vi "s.vi"() -> ()   [LabVIEW 2013] (continued)
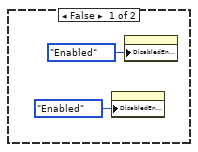
[diagram p2: hidden frame]
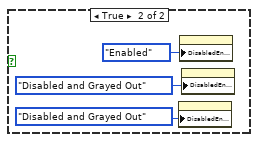
[diagram p3: hidden frame]
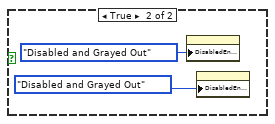
[diagram p4: hidden frame]
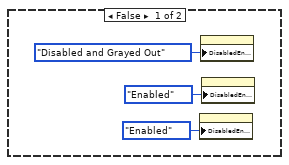
[diagram p5: hidden frame]
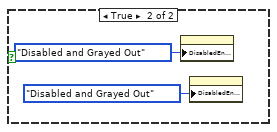
[diagram p6: hidden frame]
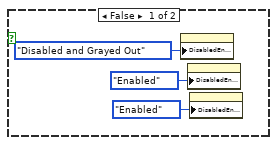
[diagram p7: hidden frame]
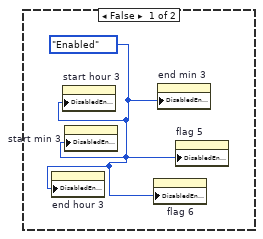
[diagram p8: hidden frame]
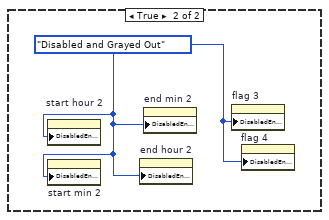
[diagram p9: hidden frame]
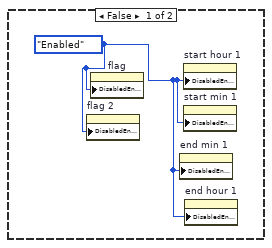
[diagram p10: hidden frame]
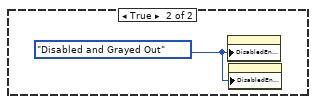
[diagram p11: hidden frame]
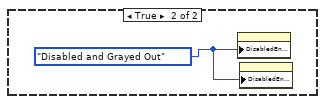
[diagram p12: hidden frame]
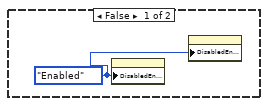
[diagram p13: hidden frame]
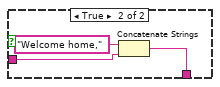
[diagram p16: hidden frame]
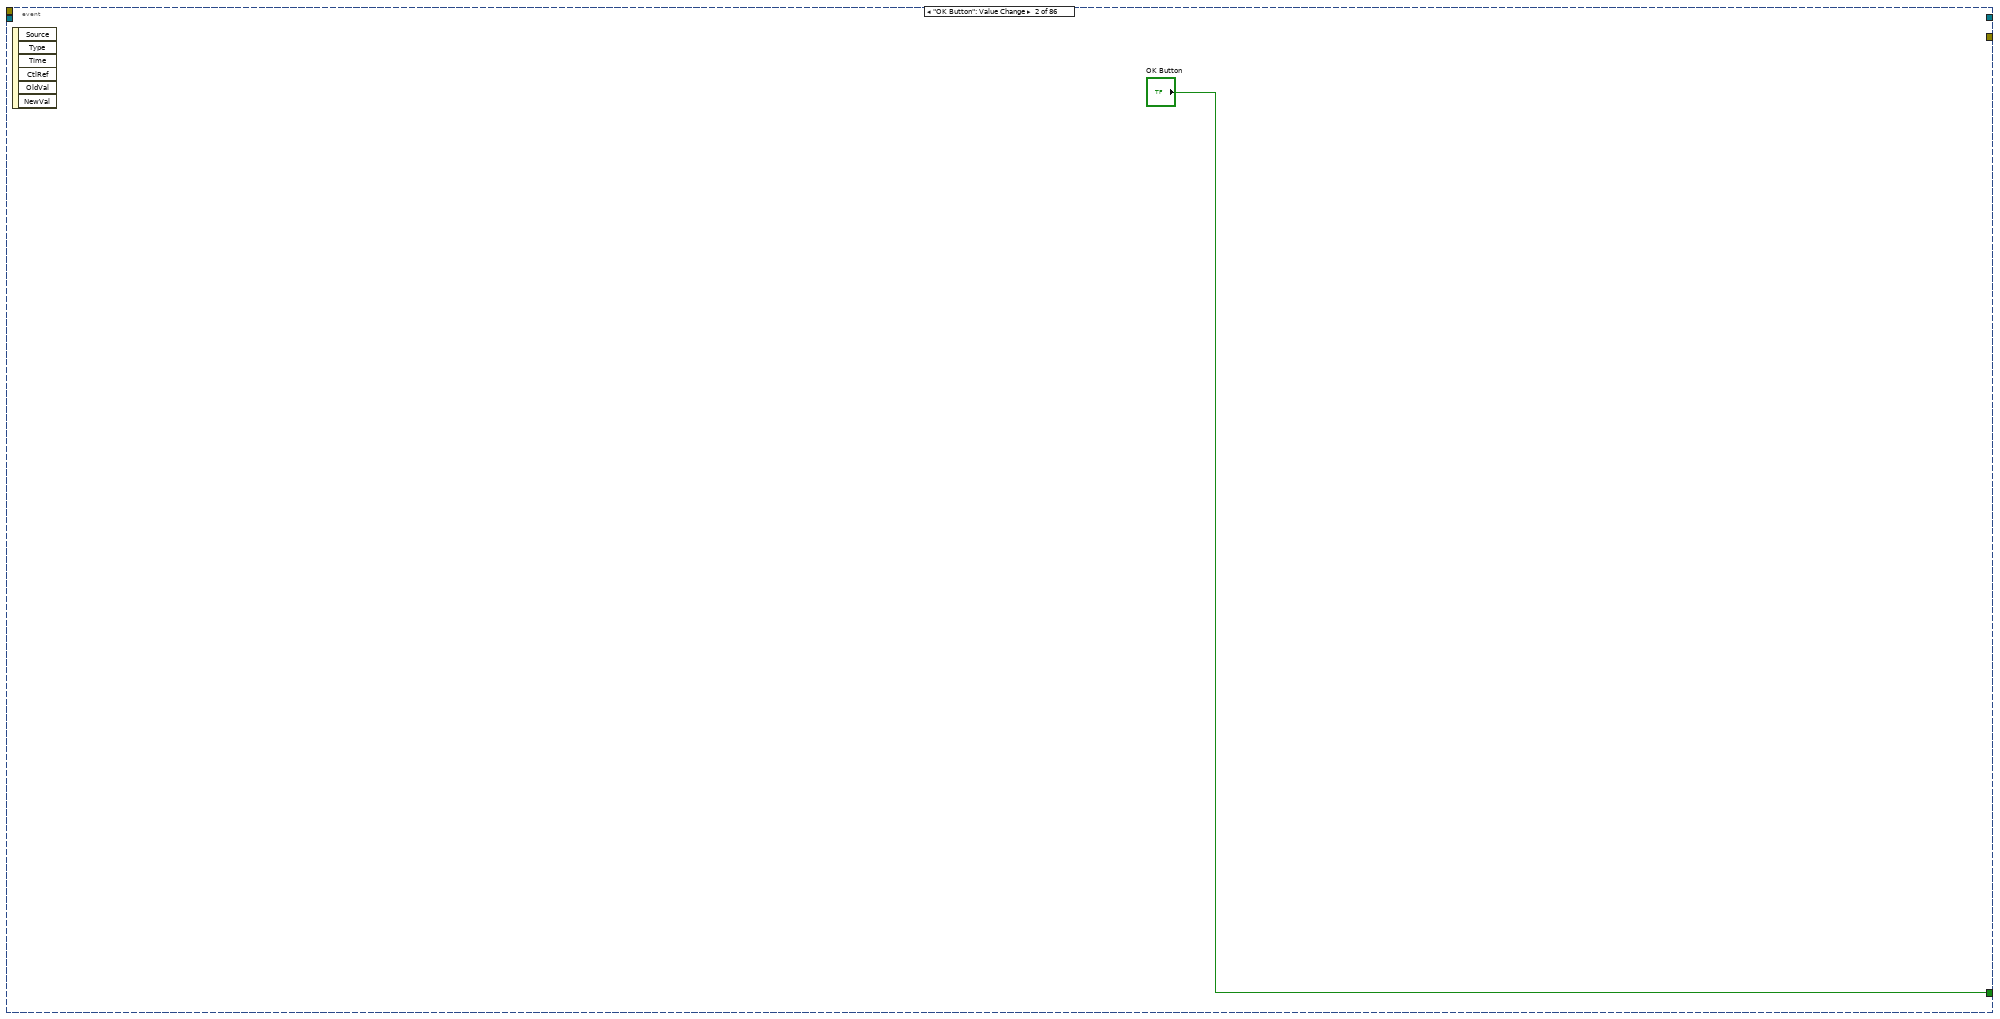
[diagram p17: hidden frame]
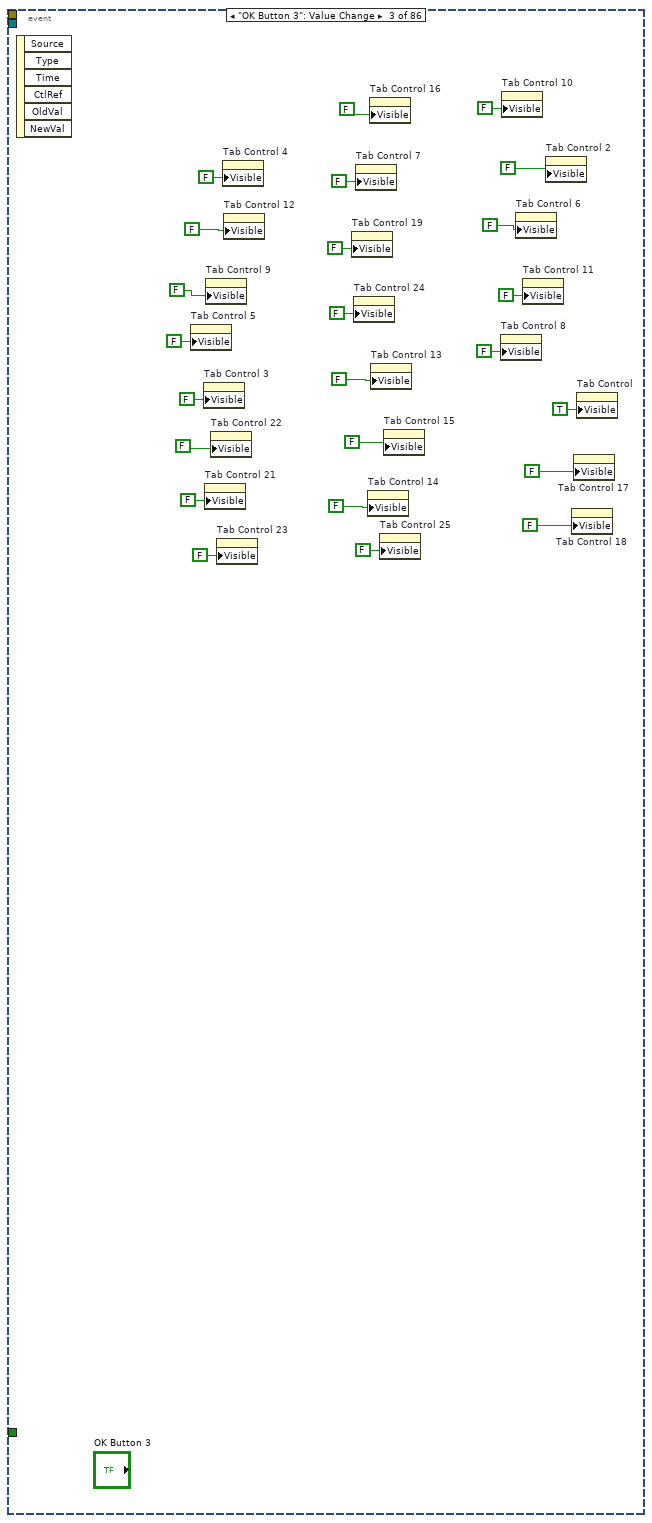
[diagram p18: hidden frame]
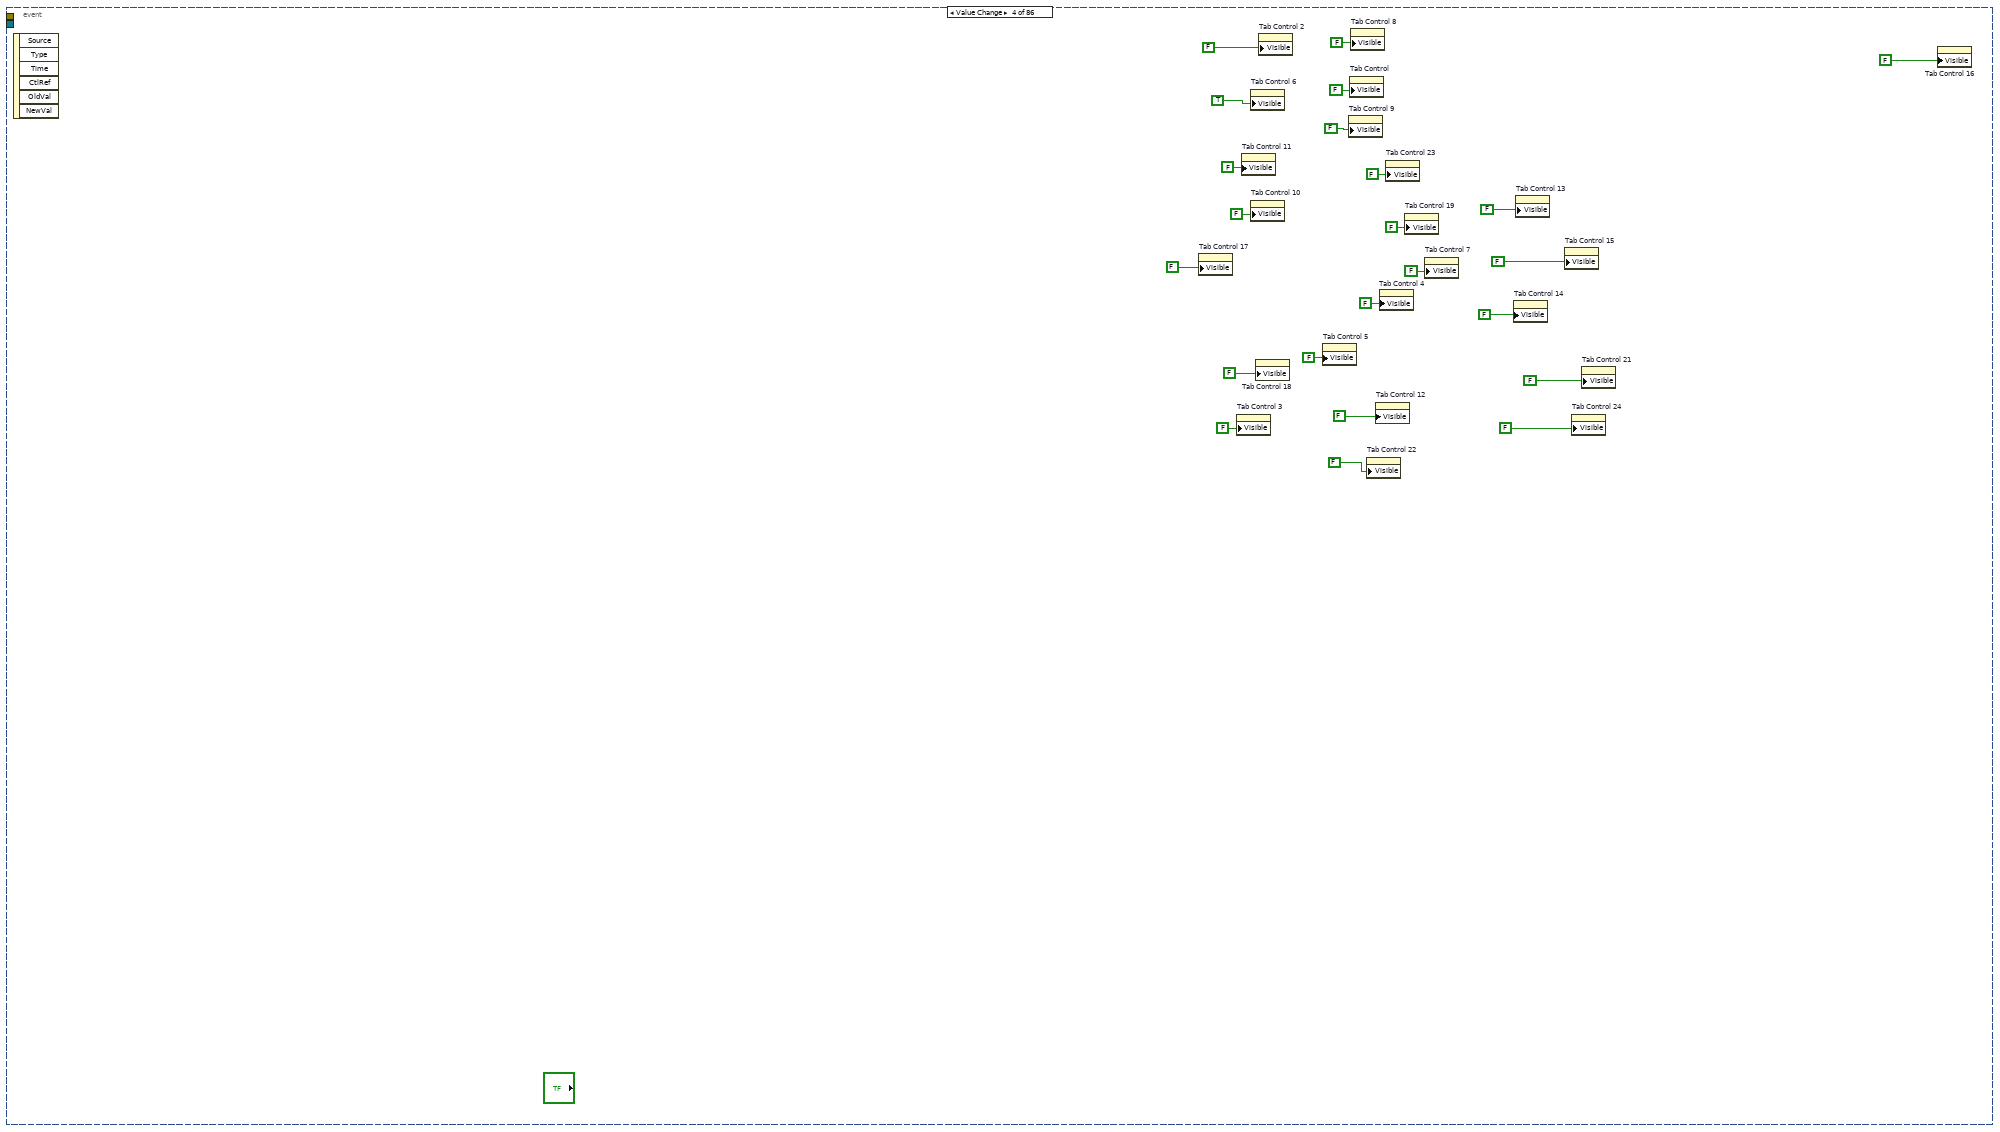
[diagram p19: hidden frame]
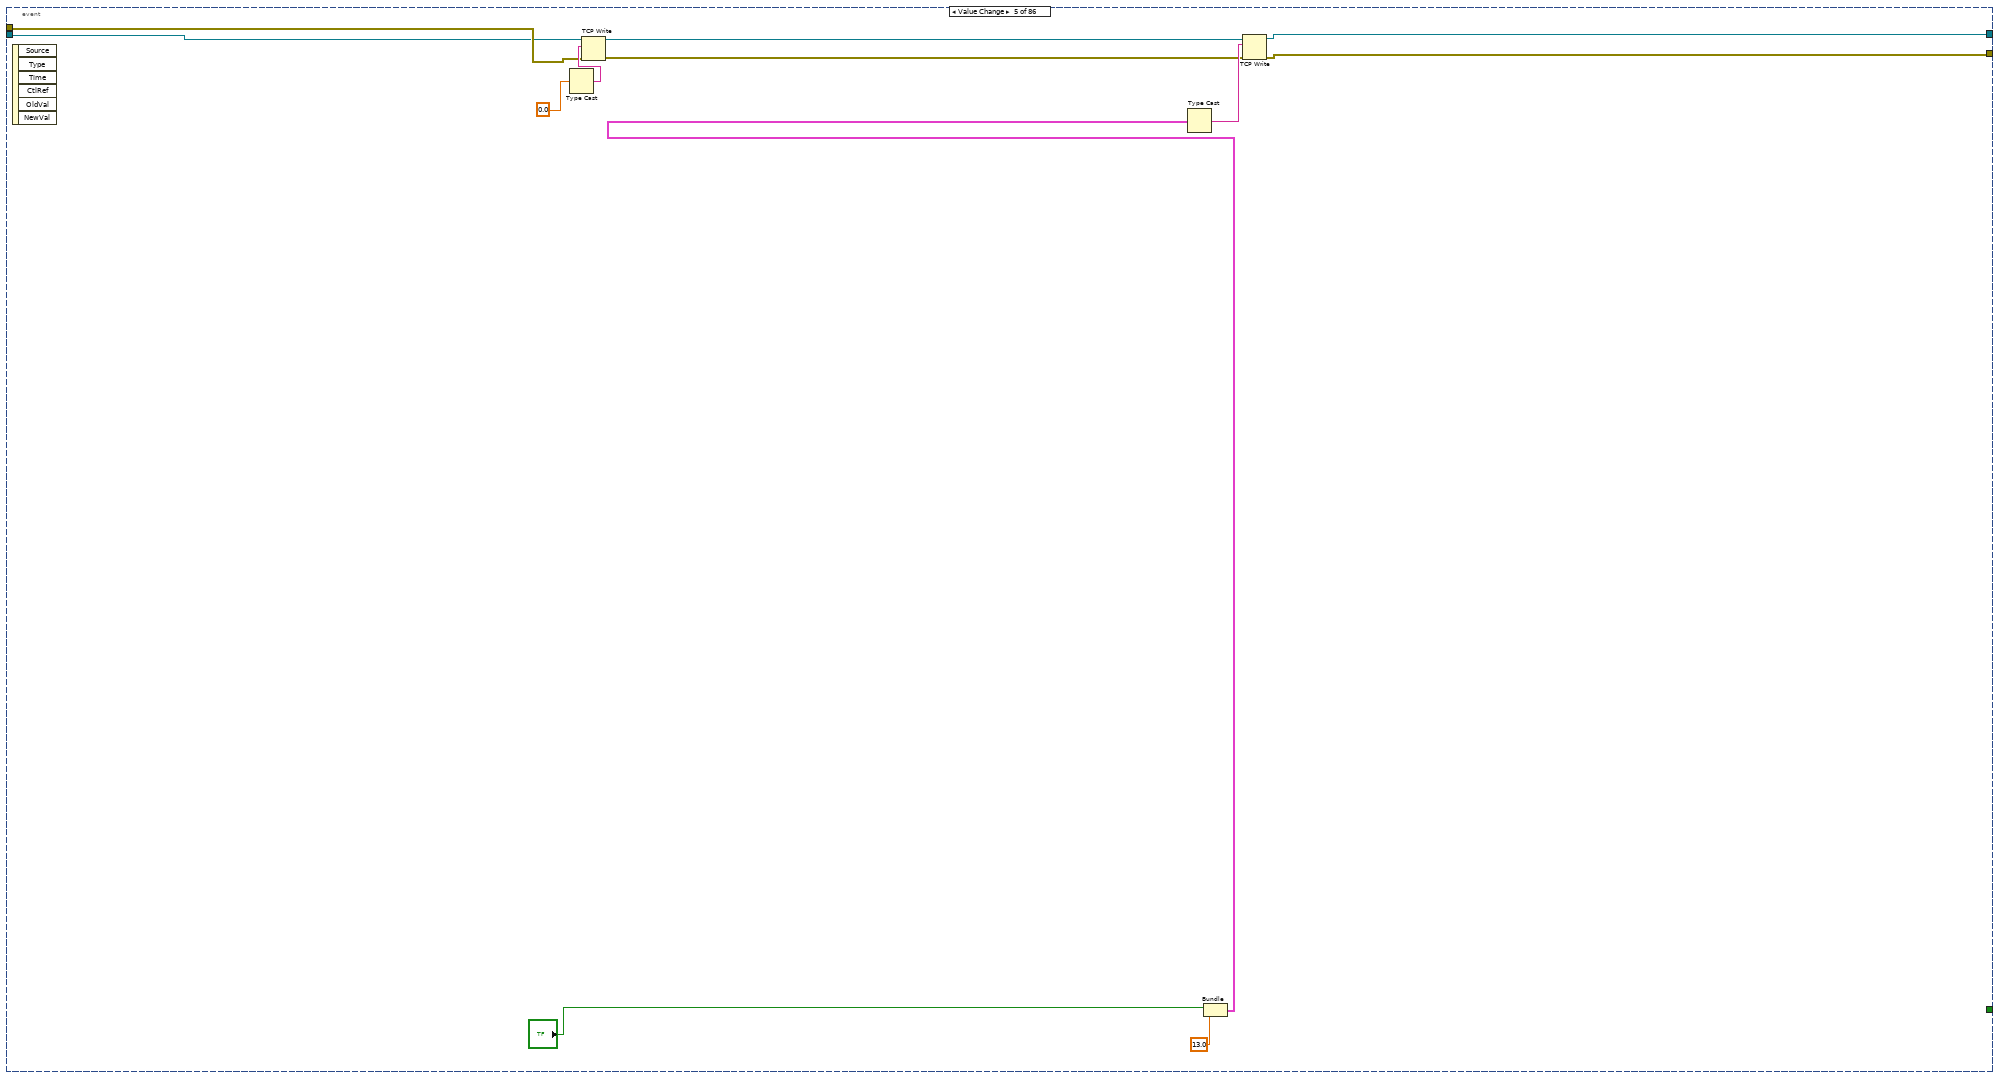
[diagram p20: hidden frame]
        n991 = property on="Tab Control 15" class="TabCtl (strict)"("Visible"=FALSE) -> ()  [unwired: 2 in, 2 out]
        n992 = property on="Tab Control 16" class="TabCtl (strict)"("Visible"=FALSE) -> ()  [unwired: 2 in, 2 out]
        n993 = property on="Tab Control 17" class="TabCtl (strict)"("Visible"=FALSE) -> ()  [unwired: 2 in, 2 out]
        n994 = property on="Tab Control 21" class="TabCtl (strict)"("Visible"=FALSE) -> ()  [unwired: 2 in, 2 out]
        n995 = property on="Tab Control 18" class="TabCtl (strict)"("Visible"=FALSE) -> ()  [unwired: 2 in, 2 out]
        n996 = property on="Tab Control 24" class="TabCtl (strict)"("Visible"=FALSE) -> ()  [unwired: 2 in, 2 out]
        n997 = property on="Tab Control 19" class="TabCtl (strict)"("Visible"=TRUE) -> ()  [unwired: 2 in, 2 out]
        n998 = property on="Tab Control 22" class="TabCtl (strict)"("Visible"=FALSE) -> ()  [unwired: 2 in, 2 out]
      }
      event "OK Button 6": Value Change {
        n999 = event-data() -> ()  [unwired: 1 in, 6 out]
        n1000 = Type Cast(x=0.0) -> (*(type *) &x=w3067:string)  [unwired: 1 in]
        n1001 = TCP Write(connection ID=w3065, data in=w3067, error in (no error)=w3066) -> (connection ID out=w3064:refnum<k5>, error out=w3063:errorcluster)  [unwired: 1 in, 1 out]
        n1002 = Bundle("OK Button 6"="OK Button 6", 5.0) -> (w3072:cluster{"OK Button 6":bool, dbl})  [unwired: 1 in]
        n1003 = Type Cast(x=w3072) -> (*(type *) &x=w3073:string)  [unwired: 1 in]
        n1004 = TCP Write(connection ID=w3064, data in=w3073, error in (no error)=w3063) -> (connection ID out=w3069:refnum<k5>, error out=w3070:errorcluster)  [unwired: 1 in, 1 out]
      }
      event Value Change {
        # "Air conditional - Master room"
        n1005 = event-data() -> ()  [unwired: 1 in, 6 out]
        n1006 = property on="Tab Control" class="TabCtl (strict)"("Visible"=FALSE) -> ()  [unwired: 2 in, 2 out]
        n1007 = property on="Tab Control 2" class="TabCtl (strict)"("Visible"=FALSE) -> ()  [unwired: 2 in, 2 out]
        n1008 = property on="Tab Control 3" class="TabCtl (strict)"("Visible"=FALSE) -> ()  [unwired: 2 in, 2 out]
        n1009 = property on="Tab Control 4" class="TabCtl (strict)"("Visible"=FALSE) -> ()  [unwired: 2 in, 2 out]
        n1010 = property on="Tab Control 5" class="TabCtl (strict)"("Visible"=FALSE) -> ()  [unwired: 2 in, 2 out]
        n1011 = property on="Tab Control 13" class="TabCtl (strict)"("Visible"=FALSE) -> ()  [unwired: 2 in, 2 out]
        n1012 = property on="Tab Control 14" class="TabCtl (strict)"("Visible"=FALSE) -> ()  [unwired: 2 in, 2 out]
        n1013 = property on="Tab Control 11" class="TabCtl (strict)"("Visible"=FALSE) -> ()  [unwired: 2 in, 2 out]
        n1014 = property on="Tab Control 6" class="TabCtl (strict)"("Visible"=FALSE) -> ()  [unwired: 2 in, 2 out]
        n1015 = property on="Tab Control 10" class="TabCtl (strict)"("Visible"=FALSE) -> ()  [unwired: 2 in, 2 out]
        n1016 = property on="Tab Control 7" class="TabCtl (strict)"("Visible"=FALSE) -> ()  [unwired: 2 in, 2 out]
        n1017 = property on="Tab Control 12" class="TabCtl (strict)"("Visible"=FALSE) -> ()  [unwired: 2 in, 2 out]
        n1018 = property on="Tab Control 8" class="TabCtl (strict)"("Visible"=FALSE) -> ()  [unwired: 2 in, 2 out]
        n1019 = property on="Tab Control 9" class="TabCtl (strict)"("Visible"=FALSE) -> ()  [unwired: 2 in, 2 out]
        n1020 = property on="Tab Control 15" class="TabCtl (strict)"("Visible"=FALSE) -> ()  [unwired: 2 in, 2 out]
        n1021 = property on="Tab Control 16" class="TabCtl (strict)"("Visible"=FALSE) -> ()  [unwired: 2 in, 2 out]
        n1022 = property on="Tab Control 17" class="TabCtl (strict)"("Visible"=FALSE) -> ()  [unwired: 2 in, 2 out]
        n1023 = property on="Tab Control 24" class="TabCtl (strict)"("Visible"=FALSE) -> ()  [unwired: 2 in, 2 out]
        n1024 = property on="Tab Control 18" class="TabCtl (strict)"("Visible"=FALSE) -> ()  [unwired: 2 in, 2 out]
        n1025 = property on="Tab Control 21" class="TabCtl (strict)"("Visible"=FALSE) -> ()  [unwired: 2 in, 2 out]
        n1026 = property on="Tab Control 19" class="TabCtl (strict)"("Visible"=FALSE) -> ()  [unwired: 2 in, 2 out]
        n1027 = property on="Tab Control 22" class="TabCtl (strict)"("Visible"=TRUE) -> ()  [unwired: 2 in, 2 out]
      }
      event Value Change {
        # "Air conditional - Bedroom 1"
        n1028 = event-data() -> ()  [unwired: 1 in, 6 out]
        n1029 = property on="Tab Control" class="TabCtl (strict)"("Visible"=FALSE) -> ()  [unwired: 2 in, 2 out]
        n1030 = property on="Tab Control 2" class="TabCtl (strict)"("Visible"=FALSE) -> ()  [unwired: 2 in, 2 out]
        n1031 = property on="Tab Control 3" class="TabCtl (strict)"("Visible"=FALSE) -> ()  [unwired: 2 in, 2 out]
        n1032 = property on="Tab Control 4" class="TabCtl (strict)"("Visible"=FALSE) -> ()  [unwired: 2 in, 2 out]
        n1033 = property on="Tab Control 5" class="TabCtl (strict)"("Visible"=FALSE) -> ()  [unwired: 2 in, 2 out]
        n1034 = property on="Tab Control 11" class="TabCtl (strict)"("Visible"=FALSE) -> ()  [unwired: 2 in, 2 out]
        n1035 = property on="Tab Control 6" class="TabCtl (strict)"("Visible"=FALSE) -> ()  [unwired: 2 in, 2 out]
        n1036 = property on="Tab Control 10" class="TabCtl (strict)"("Visible"=FALSE) -> ()  [unwired: 2 in, 2 out]
        n1037 = property on="Tab Control 13" class="TabCtl (strict)"("Visible"=FALSE) -> ()  [unwired: 2 in, 2 out]
        n1038 = property on="Tab Control 7" class="TabCtl (strict)"("Visible"=FALSE) -> ()  [unwired: 2 in, 2 out]
        n1039 = property on="Tab Control 12" class="TabCtl (strict)"("Visible"=FALSE) -> ()  [unwired: 2 in, 2 out]
        n1040 = property on="Tab Control 8" class="TabCtl (strict)"("Visible"=FALSE) -> ()  [unwired: 2 in, 2 out]
        n1041 = property on="Tab Control 9" class="TabCtl (strict)"("Visible"=FALSE) -> ()  [unwired: 2 in, 2 out]
        n1042 = property on="Tab Control 21" class="TabCtl (strict)"("Visible"=FALSE) -> ()  [unwired: 2 in, 2 out]
        n1043 = property on="Tab Control 22" class="TabCtl (strict)"("Visible"=FALSE) -> ()  [unwired: 2 in, 2 out]
        n1044 = property on="Tab Control 23" class="TabCtl (strict)"("Visible"=TRUE) -> ()  [unwired: 2 in, 2 out]
        n1045 = property on="Tab Control 24" class="TabCtl (strict)"("Visible"=FALSE) -> ()  [unwired: 2 in, 2 out]
        n1046 = property on="Tab Control 14" class="TabCtl (strict)"("Visible"=FALSE) -> ()  [unwired: 2 in, 2 out]
        n1047 = property on="Tab Control 15" class="TabCtl (strict)"("Visible"=FALSE) -> ()  [unwired: 2 in, 2 out]
        n1048 = property on="Tab Control 20" class="TabCtl (strict)"("Visible"=FALSE) -> ()  [unwired: 2 in, 2 out]
        n1049 = property on="Tab Control 16" class="TabCtl (strict)"("Visible"=FALSE) -> ()  [unwired: 2 in, 2 out]
        n1050 = property on="Tab Control 17" class="TabCtl (strict)"("Visible"=FALSE) -> ()  [unwired: 2 in, 2 out]
        n1051 = property on="Tab Control 18" class="TabCtl (strict)"("Visible"=FALSE) -> ()  [unwired: 2 in, 2 out]
        n1052 = property on="Tab Control 19" class="TabCtl (strict)"("Visible"=FALSE) -> ()  [unwired: 2 in, 2 out]
      }
      event "OK Button 7": Value Change {
        n1053 = event-data() -> ()  [unwired: 1 in, 6 out]
        n1054 = Type Cast(x=0.0) -> (*(type *) &x=w3125:string)  [unwired: 1 in]
        n1055 = TCP Write(connection ID=w3123, data in=w3125, error in (no error)=w3120) -> (connection ID out=w3122:refnum<k5>, error out=w3121:errorcluster)  [unwired: 1 in, 1 out]
        n1056 = Bundle("OK Button 7"="OK Button 7", 6.0) -> (w3130:cluster{"OK Button 7":bool, dbl})  [unwired: 1 in]
        n1057 = Type Cast(x=w3130) -> (*(type *) &x=w3131:string)  [unwired: 1 in]
        n1058 = TCP Write(connection ID=w3122, data in=w3131, error in (no error)=w3121) -> (connection ID out=w3127:refnum<k5>, error out=w3128:errorcluster)  [unwired: 1 in, 1 out]
      }
      event "OK Button 8": Value Change {
        n1059 = event-data() -> ()  [unwired: 1 in, 6 out]
        n1060 = Type Cast(x=0.0) -> (*(type *) &x=w3137:string)  [unwired: 1 in]
        n1061 = TCP Write(connection ID=w3133, data in=w3137, error in (no error)=w3132) -> (connection ID out=w3134:refnum<k5>, error out=w3135:errorcluster)  [unwired: 1 in, 1 out]
        n1062 = Bundle("OK Button 8"="OK Button 8", 7.0) -> (w3142:cluster{"OK Button 8":bool, dbl})  [unwired: 1 in]
        n1063 = Type Cast(x=w3142) -> (*(type *) &x=w3143:string)  [unwired: 1 in]
        n1064 = TCP Write(connection ID=w3134, data in=w3143, error in (no error)=w3135) -> (connection ID out=w3139:refnum<k5>, error out=w3140:errorcluster)  [unwired: 1 in, 1 out]
      }
      event "OK Button 9": Value Change {
        n1065 = event-data() -> ()  [unwired: 1 in, 6 out]
        n1066 = Type Cast(x=0.0) -> ()  [unwired: 1 in, 1 out]
        n1067 = TCP Write(connection ID=w3145, error in (no error)=w3144) -> (connection ID out=w3146:refnum<k5>, error out=w3147:errorcluster)  [unwired: 2 in, 1 out]
        n1068 = Bundle("OK Button 9"="OK Button 9", 10.0) -> (w3153:cluster{"OK Button 9":bool, dbl})  [unwired: 1 in]
        n1069 = Type Cast(x=w3153) -> (*(type *) &x=w3154:string)  [unwired: 1 in]
        n1070 = TCP Write(connection ID=w3146, data in=w3154, error in (no error)=w3147) -> (connection ID out=w3150:refnum<k5>, error out=w3151:errorcluster)  [unwired: 1 in, 1 out]
      }
      event "OK Button 10": Value Change {
        n1071 = event-data() -> ()  [unwired: 1 in, 6 out]
        n1072 = Type Cast(x=0.0) -> ()  [unwired: 1 in, 1 out]
        n1073 = TCP Write(connection ID=w3158, error in (no error)=w3157) -> (connection ID out=w3156:refnum<k5>, error out=w3155:errorcluster)  [unwired: 2 in, 1 out]
        n1074 = Bundle("OK Button 10"="OK Button 10", 11.0) -> (w3164:cluster{"OK Button 10":bool, dbl})  [unwired: 1 in]
        n1075 = Type Cast(x=w3164) -> (*(type *) &x=w3165:string)  [unwired: 1 in]
        n1076 = TCP Write(connection ID=w3156, data in=w3165, error in (no error)=w3155) -> (connection ID out=w3161:refnum<k5>, error out=w3162:errorcluster)  [unwired: 1 in, 1 out]
      }
    }
    n1077 = case shown="True" w28 {
      frame False {
        w75 = T1."Enabled" ("Disabled")
        n1078 = property class="Slide (strict)"("DisabledEnum"=w75) -> ()  [unwired: 2 in, 2 out]
        n1079 = property class="Str"("DisabledEnum"=w75) -> ()  [unwired: 2 in, 2 out]
      }
      frame True {
        w76 = T1."Disabled and Grayed Out" ("Disabled")
        n1080 = property class="Slide (strict)"("DisabledEnum"=w76) -> ()  [unwired: 2 in, 2 out]
        n1081 = property class="Str"("DisabledEnum"=w76) -> ()  [unwired: 2 in, 2 out]
      }
    }
    n1082 = case shown="False" w27 {
      frame False {
        w73 = T1."Enabled" ("Disabled")
        n1083 = property class="Slide (strict)"("DisabledEnum"=w73) -> ()  [unwired: 2 in, 2 out]
        n1084 = property class="Str"("DisabledEnum"=w73) -> ()  [unwired: 2 in, 2 out]
      }
      frame True {
        w74 = T1."Disabled and Grayed Out" ("Disabled")
        n1085 = property class="Slide (strict)"("DisabledEnum"=w74) -> ()  [unwired: 2 in, 2 out]
        n1086 = property class="Str"("DisabledEnum"=w74) -> ()  [unwired: 2 in, 2 out]
      }
    }
    n1087 = case shown="True" w25 {
      frame False {
        w69 = T1."Enabled" ("Disabled")
        n1088 = property on="flag 2" class="Ring (strict)"("DisabledEnum"=w69) -> ()  [unwired: 2 in, 2 out]
        n1089 = property on="flag" class="Ring (strict)"("DisabledEnum"=w69) -> ()  [unwired: 2 in, 2 out]
        n1090 = property on="end min 1" class="Ring (strict)"("DisabledEnum"=w69) -> ()  [unwired: 2 in, 2 out]
        n1091 = property on="start hour 1" class="Ring (strict)"("DisabledEnum"=w69) -> ()  [unwired: 2 in, 2 out]
        n1092 = property on="start min 1" class="Ring (strict)"("DisabledEnum"=w69) -> ()  [unwired: 2 in, 2 out]
        n1093 = property on="end hour 1" class="Ring (strict)"("DisabledEnum"=w69) -> ()  [unwired: 2 in, 2 out]
      }
      frame True {
        w70 = T1."Disabled and Grayed Out" ("Disabled")
        n1094 = property on="flag 2" class="Ring (strict)"("DisabledEnum"=w70) -> ()  [unwired: 2 in, 2 out]
        n1095 = property on="flag" class="Ring (strict)"("DisabledEnum"=w70) -> ()  [unwired: 2 in, 2 out]
        n1096 = property on="end min 1" class="Ring (strict)"("DisabledEnum"=w70) -> ()  [unwired: 2 in, 2 out]
        n1097 = property on="start hour 1" class="Ring (strict)"("DisabledEnum"=w70) -> ()  [unwired: 2 in, 2 out]
        n1098 = property on="start min 1" class="Ring (strict)"("DisabledEnum"=w70) -> ()  [unwired: 2 in, 2 out]
        n1099 = property on="end hour 1" class="Ring (strict)"("DisabledEnum"=w70) -> ()  [unwired: 2 in, 2 out]
      }
    }
    n1100 = case shown="False" w26 {
      frame False {
        w71 = T1."Enabled" ("Disabled")
        n1101 = property class="Slide (strict)"("DisabledEnum"=w71) -> ()  [unwired: 2 in, 2 out]
        n1102 = property class="Str"("DisabledEnum"=w71) -> ()  [unwired: 2 in, 2 out]
      }
      frame True {
        w72 = T1."Disabled and Grayed Out" ("Disabled")
        n1103 = property class="Slide (strict)"("DisabledEnum"=w72) -> ()  [unwired: 2 in, 2 out]
        n1104 = property class="Str"("DisabledEnum"=w72) -> ()  [unwired: 2 in, 2 out]
      }
    }
    n1105 = case shown="False" w24 {
      frame False {
        w67 = T1."Enabled" ("Disabled")
        n1106 = property on="start hour 2" class="Ring (strict)"("DisabledEnum"=w67) -> ()  [unwired: 2 in, 2 out]
        n1107 = property on="start min 2" class="Ring (strict)"("DisabledEnum"=w67) -> ()  [unwired: 2 in, 2 out]
        n1108 = property on="end hour 2" class="Ring (strict)"("DisabledEnum"=w67) -> ()  [unwired: 2 in, 2 out]
        n1109 = property on="end min 2" class="Ring (strict)"("DisabledEnum"=w67) -> ()  [unwired: 2 in, 2 out]
        n1110 = property on="flag 3" class="Ring (strict)"("DisabledEnum"=w67) -> ()  [unwired: 2 in, 2 out]
        n1111 = property on="flag 4" class="Ring (strict)"("DisabledEnum"=w67) -> ()  [unwired: 2 in, 2 out]
      }
      frame True {
        w68 = T1."Disabled and Grayed Out" ("Disabled")
        n1112 = property on="start hour 2" class="Ring (strict)"("DisabledEnum"=w68) -> ()  [unwired: 2 in, 2 out]
        n1113 = property on="start min 2" class="Ring (strict)"("DisabledEnum"=w68) -> ()  [unwired: 2 in, 2 out]
        n1114 = property on="end hour 2" class="Ring (strict)"("DisabledEnum"=w68) -> ()  [unwired: 2 in, 2 out]
        n1115 = property on="end min 2" class="Ring (strict)"("DisabledEnum"=w68) -> ()  [unwired: 2 in, 2 out]
        n1116 = property on="flag 3" class="Ring (strict)"("DisabledEnum"=w68) -> ()  [unwired: 2 in, 2 out]
        n1117 = property on="flag 4" class="Ring (strict)"("DisabledEnum"=w68) -> ()  [unwired: 2 in, 2 out]
      }
    }
    n1118 = case shown="True" w23 {
      frame False {
        w65 = T1."Enabled" ("Disabled")
        n1119 = property on="end hour 3" class="Ring (strict)"("DisabledEnum"=w65) -> ()  [unwired: 2 in, 2 out]
        n1120 = property on="start hour 3" class="Ring (strict)"("DisabledEnum"=w65) -> ()  [unwired: 2 in, 2 out]
        n1121 = property on="start min 3" class="Ring (strict)"("DisabledEnum"=w65) -> ()  [unwired: 2 in, 2 out]
        n1122 = property on="flag 6" class="Ring (strict)"("DisabledEnum"=w65) -> ()  [unwired: 2 in, 2 out]
        n1123 = property on="end min 3" class="Ring (strict)"("DisabledEnum"=w65) -> ()  [unwired: 2 in, 2 out]
        n1124 = property on="flag 5" class="Ring (strict)"("DisabledEnum"=w65) -> ()  [unwired: 2 in, 2 out]
      }
      frame True {
        w66 = T1."Disabled and Grayed Out" ("Disabled")
        n1125 = property on="end hour 3" class="Ring (strict)"("DisabledEnum"=w66) -> ()  [unwired: 2 in, 2 out]
        n1126 = property on="start hour 3" class="Ring (strict)"("DisabledEnum"=w66) -> ()  [unwired: 2 in, 2 out]
        n1127 = property on="start min 3" class="Ring (strict)"("DisabledEnum"=w66) -> ()  [unwired: 2 in, 2 out]
        n1128 = property on="flag 6" class="Ring (strict)"("DisabledEnum"=w66) -> ()  [unwired: 2 in, 2 out]
        n1129 = property on="end min 3" class="Ring (strict)"("DisabledEnum"=w66) -> ()  [unwired: 2 in, 2 out]
        n1130 = property on="flag 5" class="Ring (strict)"("DisabledEnum"=w66) -> ()  [unwired: 2 in, 2 out]
      }
    }
    n1131 = case shown="True" w34 {
      frame False {
      }
      frame True {
        n1132 = Read from Text File(file (use dialog)=path "C:/Users/kiat/Desktop/password.txt") -> (text=w77:string)  [unwired: 3 in, 3 out]
        n1133 = while {
          border: w77 -> [_]
          stop <- TRUE stop-if-true
          (unwired) "\n"
          n1134 = feedback #7() -> (w89:string)
          n1135 = xnode "Match Regular Expression"("input string"=w89, "regular expression"="\n") -> ("before match"=w87:string, "after match"=w88:string)  [unwired: 4 in, 3 out]
          n1136 = feedback-in #7(w88) -> ()
          n1137 = xnode "Match Regular Expression"("input string"=w87, "regular expression"="-") -> ("before match"=w98:string, "after match"=w86:string)  [unwired: 4 in, 3 out]
          n1138 = xnode "Match Regular Expression"("input string"=w86, "regular expression"=":") -> ("before match"=w84:string, "after match"=w83:string)  [unwired: 4 in, 3 out]
          n1139 = Equal?(x=w83, y="Admin") -> (x = y?=w81:bool)
          n1140 = Equal?(x="String", y=w98) -> (x = y?=w95:bool)
          n1141 = Equal?(x=w84, y="String 2") -> (x = y?=w96:bool)
          n1142 = And(x=w95, y=w96) -> (x .and. y?=w79:bool)
          n1143 = And(x=w79, y=w81) -> (x .and. y?=w80:bool)
          n1144 = case shown="False" w79 {
            tunnel: "String" -> [_ w332]
            tunnel: ["Access deneid." w331] -> w93
            frame False {
            }
            frame True {
              n1145 = Concatenate Strings("Welcome home," ("string"), w332) -> (w331:string)
            }
          }
          n1146 = call "Display Message to User"("Enable"=TRUE, "Message"=w93) -> ()  [unwired: 8 in, 2 out]
          n1147 = case shown="True" w80 {
            frame False {
            }
            frame True {
              n1148 = property on="Tab Control 2" class="TabCtl (strict)"("Visible"=TRUE) -> ()  [unwired: 2 in, 2 out]
              n1149 = property on="Tab Control" class="TabCtl (strict)"("Visible"=FALSE) -> ()  [unwired: 2 in, 2 out]
            }
          }
        }
      }
    }
    n1150 = local read item#11() -> (w21:bool)
    n1151 = local read item#9() -> (w22:bool)
    n1152 = local read item#5() -> (w20:bool)
    n1153 = case shown="False" w21 {
      frame False {
        n1154 = property class="Bool (strict)"("DisabledEnum"=T1."Enabled" ("Disabled")) -> ()  [unwired: 2 in, 2 out]
        n1155 = property class="Slide (strict)"("DisabledEnum"=T1."Enabled" ("Disabled")) -> ()  [unwired: 2 in, 2 out]
      }
      frame True {
        n1156 = property class="Bool (strict)"("DisabledEnum"=T1."Disabled and Grayed Out" ("Disabled")) -> ()  [unwired: 2 in, 2 out]
        n1157 = property class="Slide (strict)"("DisabledEnum"=T1."Disabled and Grayed Out" ("Disabled")) -> ()  [unwired: 2 in, 2 out]
      }
    }
    n1158 = case shown="True" w22 {
      frame False {
        n1159 = property class="Slide (strict)"("DisabledEnum"=T1."Disabled and Grayed Out" ("Disabled")) -> ()  [unwired: 2 in, 2 out]
        n1160 = property class="Bool (strict)"("DisabledEnum"=T1."Enabled" ("Disabled")) -> ()  [unwired: 2 in, 2 out]
        n1161 = property class="Str"("DisabledEnum"=T1."Enabled" ("Disabled")) -> ()  [unwired: 2 in, 2 out]
      }
      frame True {
        n1162 = property class="Slide (strict)"("DisabledEnum"=T1."Enabled" ("Disabled")) -> ()  [unwired: 2 in, 2 out]
        n1163 = property class="Bool (strict)"("DisabledEnum"=T1."Disabled and Grayed Out" ("Disabled")) -> ()  [unwired: 2 in, 2 out]
        n1164 = property class="Str"("DisabledEnum"=T1."Disabled and Grayed Out" ("Disabled")) -> ()  [unwired: 2 in, 2 out]
      }
    }
    n1165 = case shown="True" w20 {
      frame False {
        n1166 = property class="Str"("DisabledEnum"=T1."Enabled" ("Disabled")) -> ()  [unwired: 2 in, 2 out]
        n1167 = property class="Slide (strict)"("DisabledEnum"=T1."Disabled and Grayed Out" ("Disabled")) -> ()  [unwired: 2 in, 2 out]
        n1168 = property class="Bool (strict)"("DisabledEnum"=T1."Enabled" ("Disabled")) -> ()  [unwired: 2 in, 2 out]
      }
      frame True {
        n1169 = property class="Str"("DisabledEnum"=T1."Disabled and Grayed Out" ("Disabled")) -> ()  [unwired: 2 in, 2 out]
        n1170 = property class="Slide (strict)"("DisabledEnum"=T1."Enabled" ("Disabled")) -> ()  [unwired: 2 in, 2 out]
        n1171 = property class="Bool (strict)"("DisabledEnum"=T1."Disabled and Grayed Out" ("Disabled")) -> ()  [unwired: 2 in, 2 out]
      }
    }
    n1172 = local read item#7() -> (w19:bool)
    n1173 = case shown="False" w19 {
      frame False {
        n1174 = property class="Slide (strict)"("DisabledEnum"=T1."Enabled" ("Disabled")) -> ()  [unwired: 2 in, 2 out]
        n1175 = property class="Bool (strict)"("DisabledEnum"=T1."Enabled" ("Disabled")) -> ()  [unwired: 2 in, 2 out]
      }
      frame True {
        n1176 = property class="Slide (strict)"("DisabledEnum"=T1."Disabled and Grayed Out" ("Disabled")) -> ()  [unwired: 2 in, 2 out]
        n1177 = property class="Bool (strict)"("DisabledEnum"=T1."Disabled and Grayed Out" ("Disabled")) -> ()  [unwired: 2 in, 2 out]
      }
    }
    n1178 = local read item#1() -> (w18:bool)
    n1179 = local read item#3() -> (w17:bool)
    n1180 = case shown="False" w18 {
      frame False {
        n1181 = property class="Bool (strict)"("DisabledEnum"=T1."Enabled" ("Disabled")) -> ()  [unwired: 2 in, 2 out]
        n1182 = property class="Str"("DisabledEnum"=T1."Enabled" ("Disabled")) -> ()  [unwired: 2 in, 2 out]
        n1183 = property class="Slide (strict)"("DisabledEnum"=T1."Disabled and Grayed Out" ("Disabled")) -> ()  [unwired: 2 in, 2 out]
      }
      frame True {
        n1184 = property class="Str"("DisabledEnum"=T1."Disabled and Grayed Out" ("Disabled")) -> ()  [unwired: 2 in, 2 out]
        n1185 = property class="Slide (strict)"("DisabledEnum"=T1."Enabled" ("Disabled")) -> ()  [unwired: 2 in, 2 out]
        n1186 = property class="Bool (strict)"("DisabledEnum"=T1."Disabled and Grayed Out" ("Disabled")) -> ()  [unwired: 2 in, 2 out]
      }
    }
    n1187 = case shown="True" w17 {
      frame False {
        n1188 = property class="Bool (strict)"("DisabledEnum"=T1."Enabled" ("Disabled")) -> ()  [unwired: 2 in, 2 out]
        n1189 = property class="Slide (strict)"("DisabledEnum"=T1."Enabled" ("Disabled")) -> ()  [unwired: 2 in, 2 out]
      }
      frame True {
        n1190 = property class="Bool (strict)"("DisabledEnum"=T1."Disabled and Grayed Out" ("Disabled")) -> ()  [unwired: 2 in, 2 out]
        n1191 = property class="Slide (strict)"("DisabledEnum"=T1."Disabled and Grayed Out" ("Disabled")) -> ()  [unwired: 2 in, 2 out]
      }
    }
  }
  n1192 = Read from Text File(file (use dialog)=path "C:/Users/kiat/Desktop/password.txt") -> (text=w1:string)  [unwired: 3 in, 3 out]
  n1193 = while {
    border: w1 -> [_]
    stop <- w3174 stop-if-true
    n1194 = feedback #8() -> (w3178:string)
    n1195 = xnode "Match Regular Expression"("input string"=w3178, "regular expression"="\n") -> ("before match"=w3177:string, "after match"=w3176:string)  [unwired: 4 in, 3 out]
    n1196 = feedback-in #8(w3176) -> ()
    n1197 = xnode "Match Regular Expression"("input string"=w3177, "regular expression"="-") -> ("before match"=w3173:string, "after match"=w3172:string)  [unwired: 4 in, 3 out]
    n1198 = Equal?(x=w3176, y="") -> (x = y?=w3174:bool)
    n1199 = xnode "Match Regular Expression"("input string"=w3172, "regular expression"=":") -> ("before match"=w3169:string, "after match"=w3170:string)  [unwired: 4 in, 3 out]
    n1200 = local read "Table Control"() -> (w3166:string[][])
    n1201 = Build Array(w3173, w3169, w3170) -> (w3168:string[])
    n1202 = Insert Into Array(array=w3166, new element=w3168) -> (w3167:string[][])  [unwired: 2 in]
    n1203 = local write "Table Control"(w3167) -> ()
  }
  n1204 = TCP Close Connection(connection ID=w10, error in (no error)=w7) -> (error out=w11:errorcluster)  [unwired: 1 in, 1 out]
  n1205 = call <vilib>:"Clear Errors.vi"("error in (no error)"=w11) -> ()  [unwired: 6 in, 1 out]
  "Table Control" <- string[][] [] ("Table Control")
  "Numeric" <- 1.0
